vi "LauraMod_GlueFatLines.vi"(5 "Image Feed":T6=refnum, 7 "Template Path":path=path "C:/Users/Aerotech/Documents/BNL_ThermomechanicalStave/Utils/ConfigurationFiles_and_Templates/1_ModulePlacement", 8 "error in":errorcluster, 9 "um/pix resolution":dbl=1.58, 10 "Module corner coordinates":T2={"X [mm]"=-59.42477770816987, "Y [mm]"=4.341763392096446, "Z [mm] "=36.00000100000001}, 11 "XYZ Stage Control":refnum<k24>) -> (0 "error out":errorcluster={"status"=FALSE, "code"=1073676418, "source"="VISA Close in Alyssa_GlueFatLines.vi"}, 3 "XYZ .NET Refnum out":refnum<k24>)   [LabVIEW 2016]
uses:
  C:/Users/Aerotech/Documents/BNLStaveAssembly-blueprint/Bin/Aerotech.A3200.dll
  BNLStaveAssembly-blueprint/Bin/Aerotech.A3200.dll
  <vilib>/vision/Image Controls.llb/IMAQ Image.ctl
  <vilib>/LabVIEW Interface for Arduino/Type Defs/Arduino Resource.ctl
  <vilib>/LabVIEW Interface for Arduino/Type Defs/Board Type.ctl
  Utils/Controls/All_Enums/Enum_TypeDef_TapeType.ctl
  <vilib>/LabVIEW Interface for Arduino/Type Defs/Pin Mode.ctl
  <vilib>/Analysis/coordinate.llb/2D Cartesian Coordinate Rotation (Scalar).vi
  <vilib>/LabVIEW Interface for Arduino/LabVIEW Interface for Arduino.lvlib
  <vilib>/Analysis/NI_AALPro.lvlib
panel:
  out "main line speed":cluster{dbl, dbl, dbl}={21.85792349726776, 21.85792349726776, 21.85792349726776}
  in  "?":T1(tab)
  in  "Axis speeds (mm/s)":T3={"vX [mm]"=40.0, "vY [mm]"=40.0, "vZ [mm] "=40.0}
  in  "Home?":bool
  in  "Lowest Z Position":dbl=38.0
  out "Arduino Resource":T4={"VISA resource"="GlueCTRL", "Board Type"=enum."Uno", "Connection Type"=enum."USB / Serial", "Bytes Per Packet (15)"=15}
  in  "Digital I/O Pin":u8=7
  in  "Testing?":bool
  out "Difference camera/syringe in X":dbl=-133.03368290747076
  out "Difference camera/syringe in y":dbl=-2.170984960815403
  in  "Path to save collected images":path=path "C:/Users/Aerotech/cernbox/BNL/Stave Assembly Records/2017-06-12/3"
  in  "Estimate distance y":dbl
  in  "Estimate distance x":dbl=130.0
  in  "Lowest Z position Calibration":dbl=17.0
  in  "How many lines (actual x2)":i32=7
  in  "y dist (mm)":dbl=4.5
  out "bottom line speed":cluster{dbl, dbl, dbl}={32.78688524590164, 32.78688524590164, 32.78688524590164}
  out "mid line speed":cluster{dbl, dbl, dbl}={21.85792349726776, 21.85792349726776, 21.85792349726776}
  in  "Axial?":T7
  in  "glue time":dbl=2.25 format="%#_13g"
  out "top right speed":cluster{dbl, dbl, dbl}={5.46448087431694, 5.46448087431694, 5.46448087431694}
  out "top left speed":cluster{dbl, dbl, dbl}={21.85792349726776, 21.85792349726776, 21.85792349726776}
  out "Final Position":T8={"Final X"=-59.424942872475754, "Final Y"=8.342749448838399, "Final Z"=36.000300999844}
  out "Module Start":T8={"Final X"=-59.42477770816987, "Final Y"=4.341763392096446, "Final Z"=36.00000100000001}
  # "Overview: This takes a pattern of zeroes/ones (.csv file) as well as the start coordinates of the top left corner of a module and places dots of glue  \nRequirements: NI Arduino dependencies\nInstructions: Select a .csv file (ones indicate regions for glue) as well as a starting coordinate (this is default to the top left corner of the module spacer). You \ncan also input axis speeds (default to maximum) and module lengths and widths (default to 90 mm) which are the widths of the module to which you want to \nplace glue. Lastly, one can choose to Home the stage here and can select the lowest position in Z. The default is that the stage moves down 2-3 mm in Z \nwhile dispensing.  The Arduino inputs are default and simply allow the LabView program to drigger the Arduino (which sends a signal to the dispenser). The \nprogram signals to dispense air- all other parameters such as length of dispensing (default: 350 millisec), pressure (default: 48 psi), and vacuum pressure \n(default: 7.8 psi) are set on the dispenser itself. The defaults are highly recommended here."
  # "Positioning Inputs"
  # "Arduino Inputs"
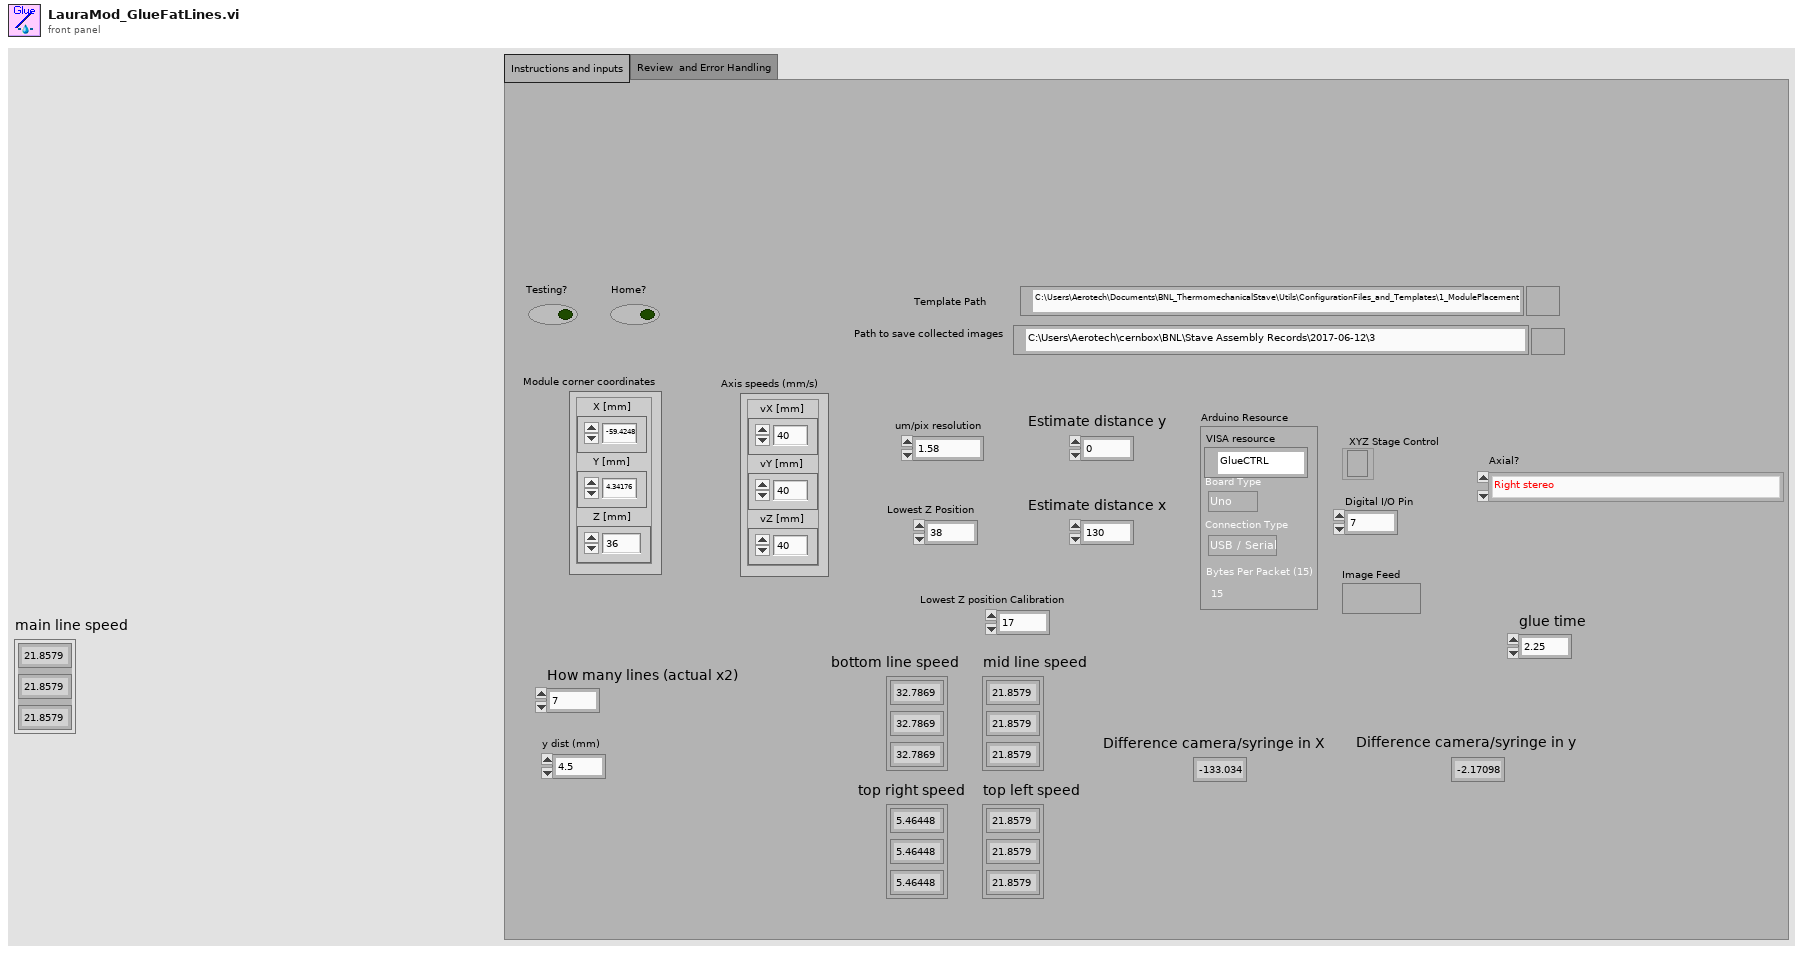
[diagram p1: front panel]
types:
  T1 = enum32{"Instructions and inputs", "Review  and Error Handling"}
  T2 = cluster{"X [mm]":dbl, "Y [mm]":dbl, "Z [mm] ":dbl}
  T3 = cluster{"vX [mm]":dbl, "vY [mm]":dbl, "vZ [mm] ":dbl}
  T4 = typedef "LabVIEW Interface for Arduino.lvlib/Arduino Resource.ctl" = cluster{"VISA resource":refnum<visa-resource-name>, "Board Type":T5, "Connection Type":enum8{"USB / Serial"}, "Bytes Per Packet (15)":u8}
  T5 = typedef "LabVIEW Interface for Arduino.lvlib/Board Type.ctl" = enum16{"Uno", "Dimuelanove w/Atmega 328", "Mega 2560"}
  T6 = typedef "IMAQ Image.ctl" = refnum<image>
  T7 = typedef "Enum_TypeDef_TapeType.ctl" = enum16{"Right stereo", "Left stereo", "Stereo (Sutcliffe Stave Core 9 LS)", "Stereo (Sutcliffe NP49-01-100 01-Mar-16)", "Stereo (Sutcliffe 21-Jun-18- Electrical)", "Axial (Sutcliffe NP49-01-100 01-Mar-16)", "Stereo (Sutcliffe Stave Core 8)"}
  T8 = cluster{"Final X":dbl, "Final Y":dbl, "Final Z":dbl}
  T9 = typedef "LabVIEW Interface for Arduino.lvlib/Pin Mode.ctl" = enum8{"Input", "Output"}
  T10 = cluster{dbl, "Y [mm]":dbl, "Lowest Z Position":dbl}
  T11 = cluster{"Final X":dbl, "Final Y":dbl, "vZ [mm]":dbl}
  T12 = cluster{dbl, "Final Y":dbl, "Lowest Z Position":dbl}
  T13 = cluster{"Final X":dbl, "Final Y":dbl, "Z [mm] ":dbl}
  T14 = cluster{"x out":dbl, "Final Y":dbl, "Lowest Z Position":dbl}
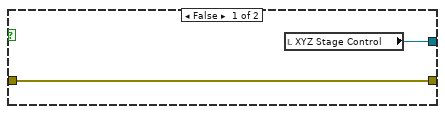
[diagram p2: hidden frame]
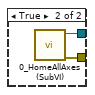
[diagram p3: hidden frame]
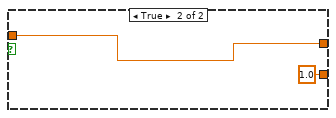
[diagram p5: hidden frame]
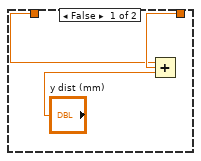
[diagram p6: hidden frame]
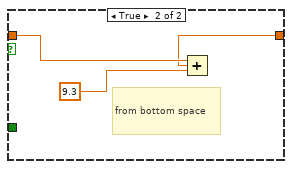
[diagram p7: hidden frame]
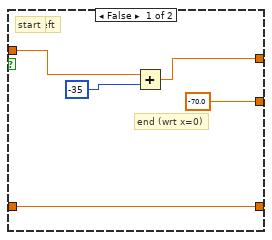
[diagram p8: hidden frame]
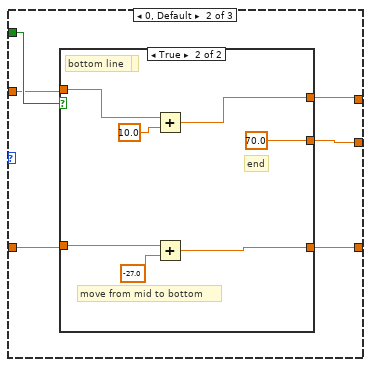
[diagram p9: hidden frame]
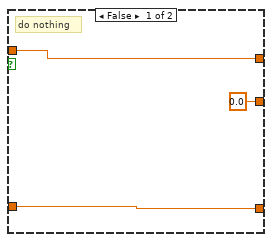
[diagram p10: hidden frame]
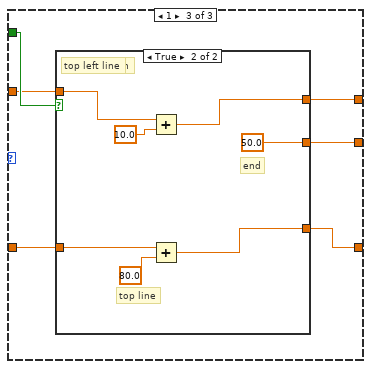
[diagram p11: hidden frame]
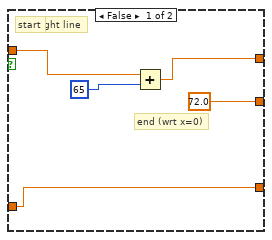
[diagram p12: hidden frame]
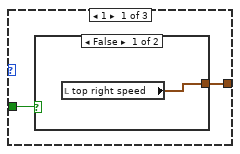
[diagram p13: hidden frame]
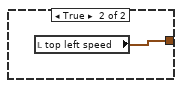
[diagram p14: hidden frame]
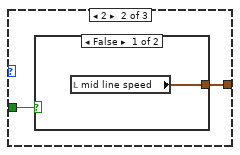
[diagram p15: hidden frame]
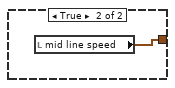
[diagram p16: hidden frame]
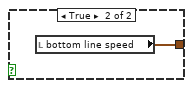
[diagram p17: hidden frame]
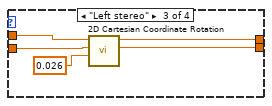
[diagram p19: hidden frame]
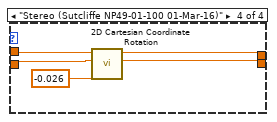
[diagram p20: hidden frame]
diagram:
  n1 = case shown="True" "Testing?" {
    tunnel: [w9 w11] -> w3
    tunnel: [w8 w10] -> w5
    tunnel: "error in" -> [w8 _]
    frame False {
      n2 = local read "XYZ Stage Control"() -> (w9:refnum<k24>)
    }
    frame True {
      n3 = case shown="False" "Home?" {
        tunnel: [w15 w21] -> w11
        tunnel: [w14 w20] -> w10
        frame False {
          w17 = string[] ["X", "Y", "Z"] ("Axes Names")
          n4 = call "Connect.vi"() -> ("error out"=w18:errorcluster, "controller"=w13:refnum<k24>)  [unwired: 10 in]
          n5 = call "EnableMultiple.vi"("error in (no error)"=w18, "axis names"=w17, "controller in"=w13) -> ("error out"=w19:errorcluster, "controller out"=w16:refnum<k24>)  [unwired: 7 in]
          n6 = call "GetCurrentXYZPosition (SubVI).vi"(".NET Refnum in - Device"=w16, "error in (no error)"=w19, "Axes Names"=w17) -> ("error out"=w14:errorcluster, ".NET Refnum out  - Device"=w15:refnum<k24>)  [unwired: 3 in, 4 out]
        }
        frame True {
          n7 = call "0_HomeAllAxes (SubVI).vi"() -> ("error out"=w20:errorcluster, "controller out"=w21:refnum<k24>)  [unwired: 8 in, 2 out]
        }
      }
    }
  }
  n8 = flat-sequence {
    tunnel: [w43] -> w7
    tunnel: w5 -> [w33]
    tunnel: w3 -> [w27]
    tunnel: [w196] -> w2
    tunnel: w7 -> [w199]
    tunnel: w2 -> [w349]
    tunnel: "Axial?" -> [w320]
    frame #0 {
      n9 = flat-sequence {
        tunnel: w33 -> [w57]
        tunnel: [w56] -> w28
        tunnel: w27 -> [w50]
        tunnel: w28 -> [w59]
        tunnel: [w58] -> w26
        tunnel: [w78] -> w30
        tunnel: w26 -> [w77]
        tunnel: w30 -> [w139]
        tunnel: [w137] -> w29
        tunnel: [w172] -> w31
        tunnel: w29 -> [w173]
        frame #0 {
          n10 = local read "Module corner coordinates"() -> (w52:T2)
          n11 = Unbundle(w52) -> ("X [mm]"=w49:dbl, "Y [mm]"=w46:dbl)  [unwired: 1 out]
          n12 = local read "Axis speeds (mm/s)"() -> (w55:T3)
          n13 = Add(x=w49, y=115.0) -> (x+y=w47:dbl)
          n14 = Bundle(w47, "Y [mm]"=w46, "Lowest Z Position"="Lowest Z Position") -> (w51:T10)  [unwired: 1 in]
          n15 = Bundle(w47, "Y [mm]"=w46, "Lowest Z Position"="Lowest Z Position") -> (w44:T10)  [unwired: 1 in]
          n16 = call "Go2XYZ (SubVI).vi"(".NET Refnum in"=w50, "Go to Coordinates"=w51, "Axis Speeds"=w55, "error in (no error)"=w57) -> (".NET Refnum out"=w54:refnum<k24>, "Final Position"=→"Final Position":T8, "error out"=w56:errorcluster)  [unwired: 7 in, 2 out]
          n17 = local write "Module corner coordinates"(w44) -> ()
          n18 = local write "XYZ Stage Control"(w54) -> ()
        }
        frame #1 {
          n19 = while {
            tunnel: w59 -> [w76]
            tunnel: [w72] -> w58
            stop <- w75 stop-if-true
            n20 = call "Lower glue mount"("error in (no error)"=w76) -> ("Move Z down"=w67:dbl, "Move Z up"=w66:dbl, "Accept current Z?"=w75:bool, "error out"=w73:errorcluster)  [unwired: 14 in, 1 out]
            n21 = local read "Module corner coordinates"() -> (w70:T2)
            n22 = local read "Lowest Z Position"() -> (w60:dbl)
            n23 = local read "Axis speeds (mm/s)"() -> (w74:T3)
            n24 = Add(x=w60, y=w67) -> (x+y=w64:dbl)
            n25 = local read "XYZ Stage Control"() -> (w62:refnum<k24>)
            n26 = Subtract(x=w64, y=w66) -> (x-y=w63:dbl)
            n27 = Unbundle(w70) -> ("X [mm]"=w69:dbl, "Y [mm]"=w68:dbl)  [unwired: 1 out]
            n28 = Bundle("X [mm]"=w69, "Y [mm]"=w68, w63) -> (w65:cluster{"X [mm]":dbl, "Y [mm]":dbl, dbl})  [unwired: 1 in]
            n29 = local write "Lowest Z Position"(w63) -> ()
            n30 = call "Go2XYZ (SubVI).vi"(".NET Refnum in"=w62, "Go to Coordinates"=w65, "Axis Speeds"=w74, "error in (no error)"=w73) -> (".NET Refnum out"=w71:refnum<k24>, "Final Position"=w61:T8, "error out"=w72:errorcluster)  [unwired: 7 in, 2 out]
            n31 = local write "Final Position"(w61) -> ()
            n32 = local write "XYZ Stage Control"(w71) -> ()
          }
        }
        frame #2 {
          n33 = call "Calibrate distance?"("error in (no error)"=w77) -> ("Calibrate distance?"=w79:bool, "error out"=w80:errorcluster)  [unwired: 16 in, 1 out]
          n34 = case shown="True" w79 {
            tunnel: w80 -> [w81 w83]
            tunnel: [w81 w84] -> w78
            frame False {
            }
            frame True {
              n35 = flat-sequence {
                tunnel: w83 -> [w86]
                tunnel: [w85] -> w82
                frame #0 {
                  n36 = local read "Final Position"() -> (w93:T8)
                  n37 = local read "Axis speeds (mm/s)"() -> (w89:T3)
                  n38 = local read "XYZ Stage Control"() -> (w88:refnum<k24>)
                  n39 = Unbundle(w93) -> ("Final X"=w91:dbl, "Final Y"=w92:dbl)  [unwired: 1 out]
                  n40 = Bundle("Final X"=w91, "Final Y"=w92, "vZ [mm]"=-20.0) -> (w95:T11)  [unwired: 1 in]
                  n41 = call "Go2XYZ (SubVI).vi"(".NET Refnum in"=w88, "Go to Coordinates"=w95, "Axis Speeds"=w89, "error in (no error)"=w86) -> (".NET Refnum out"=w87:refnum<k24>, "Final Position"=w90:T8, "error out"=w85:errorcluster)  [unwired: 7 in, 2 out]
                  n42 = local write "Final Position"(w90) -> ()
                  n43 = local write "XYZ Stage Control"(w87) -> ()
                }
              }
              n44 = while {
                tunnel: [w136] -> w84
                tunnel: w82 -> [w124]
                i -> [w121]
                stop <- w96 stop-if-true
                n45 = local read "Final Position"() -> (w98:T8)
                n46 = Unbundle(w98) -> ("Final X"=w103:dbl, "Final Y"=w101:dbl, "Final Z"=w102:dbl)
                n47 = local read "Testing?"() -> (w119:bool)
                n48 = local read "Axis speeds (mm/s)"() -> (w126:T3)
                n49 = local read "XYZ Stage Control"() -> (w122:refnum<k24>)
                n50 = Subtract(x=w101, y=220.0) -> (x-y=w99:dbl)
                n51 = Equal To 0?(x=w121) -> (x = 0?=w120:bool)
                n52 = And(x=w119, y=w120) -> (x .and. y?=w118:bool)
                n53 = Bundle("Final X"=w103, w99, "Final Z"=w102) -> (w104:cluster{"Final X":dbl, dbl, "Final Z":dbl})  [unwired: 1 in]
                n54 = call "CalibrateDistanceCameraSyringe.vi"("Path to save collected images"="Path to save collected images", "Image Feed"="Image Feed", "Off stave position"=w104, ".NET Refnum in"=w122, "Axis speeds (mm/s)"=w126, "Lowest Z Position"="Lowest Z position Calibration", "Estimate distance y"="Estimate distance y", "um/pix resolution"="um/pix resolution", "Estimate distance x"="Estimate distance x", "Template Path"="Template Path", "error in"=w124, "Testing?"=w118) -> ("XYZ .NET Refnum out"=w125:refnum<k24>, "error out"=w123:errorcluster, "X/Y difference (CAMERA - SYRINGE)"=w133:dbl[][])  [unwired: 1 in]
                n55 = local read "Difference camera/syringe in X"() -> (w108:dbl)
                n56 = local read "Difference camera/syringe in y"() -> (w105:dbl)
                n57 = local read "Lowest Z position Calibration"() -> (w110:dbl)
                n58 = call "Accept calibration?"("error in (no error)"=w123) -> ("Change in lowest Z"=w112:dbl, "Change in distance Y estimate"=w113:dbl, "Change in distance X estimate"=w114:dbl, "Accept the distance syringe/camera?"=w96:bool, "error out"=w136:errorcluster)  [unwired: 13 in, 1 out]
                n59 = local write "XYZ Stage Control"(w125) -> ()
                n60 = Index Array(array=w133, index (row) #1=0 ("index (row)"), index (col) #1=0 ("disabled index (col)"), index (row) #2=0 ("index (row)"), index (col) #2=1 ("disabled index (col)")) -> (element #1=→"Difference camera/syringe in X":dbl, element #2=→"Difference camera/syringe in y":dbl)
                n61 = Add(x=w108, y=w114) -> (x+y=w107:dbl)
                n62 = Add(x=w105, y=w113) -> (x+y=w106:dbl)
                n63 = Add(x=w110, y=w112) -> (x+y=w111:dbl)
                n64 = local write "Lowest Z position Calibration"(w111) -> ()
                n65 = local write "Difference camera/syringe in X"(w107) -> ()
                n66 = local write "Difference camera/syringe in y"(w106) -> ()
              }
            }
          }
        }
        frame #3 {
          n67 = flat-sequence {
            tunnel: w139 -> [w149]
            tunnel: [w146] -> w138
            tunnel: [w159] -> w137
            tunnel: w138 -> [w160]
            frame #0 {
              n68 = local read "Module corner coordinates"() -> (w158:T2)
              n69 = local read "Difference camera/syringe in y"() -> (w154:dbl)
              n70 = local read "Difference camera/syringe in X"() -> (w155:dbl)
              n71 = Unbundle By Name(w158) -> ("X [mm]"=w145:dbl, "Y [mm]"=w157:dbl)  [unwired: 1 out]
              n72 = Subtract(x=w157, y=w154) -> (x-y=w142:dbl)
              n73 = Subtract(x=w145, y=136.0) -> (x-y=w143:dbl)
              n74 = local read "Axis speeds (mm/s)"() -> (w150:T3)
              n75 = local read "XYZ Stage Control"() -> (w151:refnum<k24>)
              n76 = Subtract(x=w142, y=83.0) -> (x-y=w140:dbl)
              n77 = Subtract(x=w143, y=w155) -> (x-y=w156:dbl)
              n78 = Bundle(w156, w140, "index (row)"=-20.0) -> (w148:cluster{dbl, dbl, "index (row)":dbl})  [unwired: 1 in]
              n79 = call "Go2XYZ (SubVI).vi"(".NET Refnum in"=w151, "Go to Coordinates"=w148, "Axis Speeds"=w150, "error in (no error)"=w149) -> (".NET Refnum out"=w152:refnum<k24>, "Final Position"=w153:T8, "error out"=w146:errorcluster)  [unwired: 7 in, 2 out]
              n80 = local write "XYZ Stage Control"(w152) -> ()
              n81 = local write "Module corner coordinates"(w153) -> ()
            }
            frame #1 {
              n82 = local read "Module corner coordinates"() -> (w165:T2)
              n83 = local read "Lowest Z Position"() -> (w168:dbl)
              n84 = local read "Axis speeds (mm/s)"() -> (w162:T3)
              n85 = local read "XYZ Stage Control"() -> (w161:refnum<k24>)
              n86 = Unbundle(w165) -> ("X [mm]"=w166:dbl, "Y [mm]"=w167:dbl)  [unwired: 1 out]
              n87 = Subtract(x=w168, y=2.0) -> (x-y=w170:dbl)
              n88 = Bundle("X [mm]"=w166, "Y [mm]"=w167, w170) -> (w171:cluster{"X [mm]":dbl, "Y [mm]":dbl, dbl})  [unwired: 1 in]
              n89 = call "Go2XYZ (SubVI).vi"(".NET Refnum in"=w161, "Go to Coordinates"=w171, "Axis Speeds"=w162, "error in (no error)"=w160) -> (".NET Refnum out"=w163:refnum<k24>, "Final Position"=w164:T8, "error out"=w159:errorcluster)  [unwired: 7 in, 2 out]
              n90 = local write "XYZ Stage Control"(w163) -> ()
              n91 = local write "Module corner coordinates"(w164) -> ()
            }
          }
        }
        frame #4 {
          n92 = while {
            tunnel: w173 -> [w187]
            tunnel: [w189] -> w172
            stop <- w174 stop-if-true
            n93 = local read "Module corner coordinates"() -> (w186:T2)
            n94 = call "Ready to glue?"("error in (no error)"=w187) -> ("Move in Z"=w183:dbl, "Move in Y"=w184:dbl, "Move in X"=w185:dbl, "Oh yeah! Reset Arduino and go!"=w174:bool, "error out"=w188:errorcluster)  [unwired: 13 in, 1 out]
            n95 = local read "Axis speeds (mm/s)"() -> (w192:T3)
            n96 = local read "XYZ Stage Control"() -> (w190:refnum<k24>)
            n97 = Unbundle(w186) -> ("X [mm]"=w182:dbl, "Y [mm]"=w181:dbl, "Z [mm]"=w180:dbl)
            n98 = Add(x=w182, y=w185) -> (x+y=w177:dbl)
            n99 = Add(x=w181, y=w184) -> (x+y=w179:dbl)
            n100 = Add(x=w180, y=w183) -> (x+y=w178:dbl)
            n101 = Bundle(w177, w179, w178) -> (w176:cluster{dbl, dbl, dbl})  [unwired: 1 in]
            n102 = call "Go2XYZ (SubVI).vi"(".NET Refnum in"=w190, "Go to Coordinates"=w176, "Axis Speeds"=w192, "error in (no error)"=w188) -> (".NET Refnum out"=w191:refnum<k24>, "Final Position"=w175:T8, "error out"=w189:errorcluster)  [unwired: 7 in, 2 out]
            "Module Start" <- w175
            n103 = local write "Final Position"(w175) -> ()
            n104 = local write "XYZ Stage Control"(w191) -> ()
            n105 = local write "Module corner coordinates"(w175) -> ()
          }
        }
      }
      n106 = local read "Digital I/O Pin"() -> (w32:u8)
      n107 = local read "glue time"() -> (w24:dbl)
      n108 = call <vilib>:"Init.vi"("VISA resource"=refnum<visa-resource-name> "GlueCTRL", "error in"=w31) -> ("Arduino Resource"=w35:T4, "error out"=w36:errorcluster)  [unwired: 16 in]
      "Arduino Resource" <- w35
      n109 = call <vilib>:"Set Digital Pin Mode.vi"("Arduino Resource"=w35, "Digital I/O Pin"="Digital I/O Pin", "Pin Mode (Input)"=Pin_Mode."Output", "error in"=w36) -> ("Arduino Resource"=w39:T4, "error out"=w40:errorcluster)  [unwired: 10 in]
      n110 = Divide(x=80.0 ("vX [mm]"), y=w24) -> (x/y=w23:dbl)
      n111 = call <vilib>:"Digital Write Pin.vi"("Arduino Resource"=w39, "Digital I/O Pin (0)"=w32, "Value (0)"=u8 0, "error in"=w40) -> ("Arduino Resource"=w34:T4, "error out"=w43:errorcluster)  [unwired: 10 in]
      n112 = Bundle(w23, w23, w23) -> (→"main line speed":cluster{dbl, dbl, dbl})  [unwired: 1 in]
      n113 = local write "Arduino Resource"(w34) -> ()
    }
    frame #1 {
      n114 = local read "Module Start"() -> (w198:T8)
      n115 = Unbundle By Name(w198) -> ("Final X"=w193:dbl, "Final Y"=w194:dbl, "Final Z"=w197:dbl)
      n116 = for {
        N: "How many lines (actual x2)" -> [_]
        tunnel: w199 -> [w211]
        tunnel: [w210] -> w196
        shift-right: [w209] -> _
        shift-left: w194 -> [w201]
        tunnel: w197 -> [w208]
        shift-right: [w207] -> _
        shift-left: w193 -> [w202]
        i -> [w205]
        n117 = Equal?(x=w205, y=2) -> (x = y?=w203:bool)
        n118 = Equal To 0?(x=w205) -> (x = 0?=w204:bool)
        n119 = for {
          N: 2 -> [_]
          tunnel: w211 -> [w233]
          tunnel: [w231] -> w210
          shift-right: [w230] -> w209
          shift-left: w201 -> [w221]
          tunnel: w208 -> [w220]
          tunnel: w202 -> [w222]
          tunnel: [w218] -> w207
          tunnel: w204 -> [w213]
          tunnel: w203 -> [w212]
          i -> [w219]
          n120 = flat-sequence {
            tunnel: w233 -> [w251]
            tunnel: [w236] -> w228
            tunnel: [w251] -> w227
            tunnel: [w239] -> w226
            tunnel: [w238] -> w225
            tunnel: [w250] -> w224
            tunnel: [w239] -> w223
            tunnel: w222 -> [w237]
            tunnel: w221 -> [w240]
            tunnel: w220 -> [w250]
            tunnel: w219 -> [w244]
            tunnel: w213 -> [w243]
            tunnel: w212 -> [w242]
            tunnel: [w279] -> w216
            tunnel: [w280] -> w215
            tunnel: [w281] -> w214
            tunnel: w223 -> [w281]
            tunnel: w224 -> [w278]
            tunnel: w225 -> [w271]
            tunnel: w226 -> [w270]
            tunnel: w227 -> [w274]
            tunnel: w228 -> [w279]
            tunnel: [w299] -> w235
            tunnel: [w298] -> w234
            tunnel: [w297] -> w232
            tunnel: [w290] -> w229
            tunnel: w216 -> [w287]
            tunnel: w215 -> [w289]
            tunnel: w214 -> [w290]
            tunnel: [w287] -> w217
            tunnel: [w319] -> w231
            tunnel: w232 -> [w307]
            tunnel: w234 -> [w318]
            tunnel: w235 -> [w316]
            tunnel: [w306] -> w230
            tunnel: w229 -> [w306]
            tunnel: [w305] -> w218
            tunnel: w217 -> [w305]
            frame #0 {
              # "line length"
              n121 = Equal To 0?(x=w244) -> (x = 0?=w241:bool)
              n122 = case shown="False" w241 {
                tunnel: [0.0 1.0] -> w246
                tunnel: [w253 w256] -> w238
                tunnel: w237 -> [w254 w256]
                frame False {
                  # "start @ end of line"
                  n123 = Add(x=w254, y=80 ("x")) -> (x+y=w253:dbl)
                }
                frame True {
                }
              }
              n124 = And(x=w241, y=w243) -> (x .and. y?=w245:bool)
              n125 = And(x=w241, y=w242) -> (x .and. y?=w249:bool)
              n126 = case shown="False" w245 {
                tunnel: w240 -> [w259 w269]
                tunnel: [w260 w268] -> w239
                tunnel: w249 -> [w258 _]
                frame False {
                  n127 = case shown="True" w258 {
                    tunnel: [w263 w264] -> w260
                    tunnel: w259 -> [w261 w266]
                    frame False {
                      n128 = Add(x=w261, y="y dist (mm)") -> (x+y=w263:dbl)
                    }
                    frame True {
                      # "center space"
                      n129 = Add(x=w266, y=11.0) -> (x+y=w264:dbl)
                    }
                  }
                }
                frame True {
                  # "from bottom space"
                  n130 = Add(x=w269, y=9.3) -> (x+y=w268:dbl)
                }
              }
              n131 = Multiply(x=80, y=w246) -> (x*y=w247:dbl)
              n132 = Add(x=w237, y=w247) -> (x+y=w236:dbl)
            }
            frame #1 {
              n133 = local read "Axis speeds (mm/s)"() -> (w276:T3)
              n134 = local read "XYZ Stage Control"() -> (w273:refnum<k24>)
              n135 = Bundle("Final X"=w271, w270, "Final Z"=w278) -> (w277:cluster{"Final X":dbl, dbl, "Final Z":dbl})  [unwired: 1 in]
              n136 = call "Go2XYZ (SubVI).vi"(".NET Refnum in"=w273, "Go to Coordinates"=w277, "Axis Speeds"=w276, "error in (no error)"=w274) -> (".NET Refnum out"=w272:refnum<k24>, "Final Position"=w275:T8, "error out"=w280:errorcluster)  [unwired: 7 in, 2 out]
              n137 = local write "Final Position"(w275) -> ()
              n138 = local write "XYZ Stage Control"(w272) -> ()
            }
            frame #2 {
              n139 = local read "Lowest Z Position"() -> (w296:dbl)
              n140 = local read "Final Position"() -> (w291:T8)
              n141 = local read "main line speed"() -> (w286:cluster{dbl, dbl, dbl})
              n142 = Unbundle(w286) -> (w285:dbl, w284:dbl)  [unwired: 1 out]
              n143 = Bundle(w285, "x"=1.04, w284) -> (w283:cluster{dbl, "x":dbl, dbl})  [unwired: 1 in]
              n144 = local read "Arduino Resource"() -> (w300:T4)
              n145 = local read "Digital I/O Pin"() -> (w299:u8)
              n146 = Unbundle(w291) -> ("Final Y"=w288:dbl)  [unwired: 2 out]
              n147 = local read "XYZ Stage Control"() -> (w294:refnum<k24>)
              n148 = Bundle(w287, "Final Y"=w288, "Lowest Z Position"=w296) -> (w293:T12)  [unwired: 1 in]
              n149 = call "Go2XYZ (SubVI).vi"(".NET Refnum in"=w294, "Go to Coordinates"=w293, "Axis Speeds"=w283) -> (".NET Refnum out"=w295:refnum<k24>, "Final Position"=w292:T8)  [unwired: 8 in, 3 out]
              n150 = local write "Final Position"(w292) -> ()
              n151 = call <vilib>:"Digital Write Pin.vi"("Arduino Resource"=w300, "Digital I/O Pin (0)"=w299, "Value (0)"=u8 1, "error in"=w289) -> ("Arduino Resource"=w298:T4, "error out"=w297:errorcluster)  [unwired: 10 in]
              n152 = local write "Arduino Resource"(w298) -> ()
              n153 = local write "XYZ Stage Control"(w295) -> ()
            }
            frame #3 {
              n154 = local read "Final Position"() -> (w314:T8)
              n155 = local read "Module corner coordinates"() -> (w313:T2)
              n156 = call <vilib>:"Digital Write Pin.vi"("Arduino Resource"=w318, "Digital I/O Pin (0)"=w316, "Value (0)"=u8 0, "error in"=w307) -> ("Arduino Resource"=w315:T4, "error out"=w319:errorcluster)  [unwired: 10 in]
              n157 = Unbundle(w314) -> ("Final X"=w304:dbl, "Final Y"=w303:dbl)  [unwired: 1 out]
              n158 = local write "Arduino Resource"(w315) -> ()
              n159 = Unbundle(w313) -> ("Z [mm]"=w312:dbl)  [unwired: 2 out]
              n160 = local read "XYZ Stage Control"() -> (w309:refnum<k24>)
              n161 = local read "Axis speeds (mm/s)"() -> (w310:T3)
              n162 = Bundle("Final X"=w304, "Final Y"=w303, "Z [mm]"=w312) -> (w311:T13)  [unwired: 1 in]
              n163 = call "Go2XYZ (SubVI).vi"(".NET Refnum in"=w309, "Go to Coordinates"=w311, "Axis Speeds"=w310) -> (".NET Refnum out"=w302:refnum<k24>, "Final Position"=w308:T8)  [unwired: 8 in, 3 out]
              n164 = local write "Final Position"(w308) -> ()
              n165 = local write "XYZ Stage Control"(w302) -> ()
            }
          }
        }
      }
    }
    frame #2 {
      n166 = local read "glue time"() -> (w334:dbl)
      n167 = local read "Module Start"() -> (w350:T8)
      n168 = Unbundle By Name(w350) -> ("Final X"=w338:dbl, "Final Y"=w339:dbl, "Final Z"=w348:dbl)
      n169 = Divide(x=35.0 ("vX [mm]"), y=w334) -> (x/y=w332:dbl)
      n170 = Divide(x=60.0 ("vX [mm]"), y="glue time") -> (x/y=w333:dbl)
      n171 = Bundle(w332, w332, w332) -> (→"mid line speed":cluster{dbl, dbl, dbl})  [unwired: 1 in]
      n172 = Bundle(w333, w333, w333) -> (→"bottom line speed":cluster{dbl, dbl, dbl})  [unwired: 1 in]
      n173 = for {
        N: 3 -> [_]
        tunnel: w349 -> [w368]
        tunnel: [w367] -> w342
        shift-right: [w365] -> _
        shift-left: w339 -> [w366]
        tunnel: w348 -> [w364]
        shift-right: [w363] -> _
        shift-left: w338 -> [w362]
        tunnel: w320 -> [w353]
        tunnel: w320 -> [w352]
        tunnel: w320 -> [w351]
        i -> [w357]
        n174 = Equal?(x=w357, y=2) -> (x = y?=w354:bool)
        n175 = Equal?(x=w357, y=1) -> (x = y?=w355:bool)
        n176 = Equal?(x=w357, y=0) -> (x = y?=w356:bool)
        n177 = for {
          N: 2 -> [_]
          tunnel: w368 -> [w403]
          tunnel: [w401] -> w367
          shift-right: [w400] -> w365
          shift-left: w366 -> [w392]
          tunnel: w364 -> [w391]
          tunnel: w362 -> [w384]
          tunnel: [w389] -> w363
          tunnel: w356 -> [w383]
          tunnel: w355 -> [w382]
          tunnel: w354 -> [w373]
          tunnel: w353 -> [w371]
          tunnel: w352 -> [w370]
          tunnel: w351 -> [w369]
          i -> [w390]
          n178 = flat-sequence {
            tunnel: w403 -> [w418]
            tunnel: [w416] -> w398
            tunnel: [w418] -> w397
            tunnel: [w408] -> w396
            tunnel: [w409] -> w395
            tunnel: [w417] -> w394
            tunnel: [w408] -> w393
            tunnel: w384 -> [w407]
            tunnel: w392 -> [w406]
            tunnel: w391 -> [w417]
            tunnel: w390 -> [w414]
            tunnel: w383 -> [w413]
            tunnel: w382 -> [w412]
            tunnel: w373 -> [w411]
            tunnel: [w405] -> w381
            tunnel: [w404] -> w380
            tunnel: [w404] -> w374
            tunnel: [w488] -> w387
            tunnel: [w487] -> w386
            tunnel: [w486] -> w385
            tunnel: w393 -> [w486]
            tunnel: w394 -> [w485]
            tunnel: w395 -> [w479]
            tunnel: w396 -> [w478]
            tunnel: w397 -> [w482]
            tunnel: w398 -> [w488]
            tunnel: w381 -> [w474]
            tunnel: w380 -> [w473]
            tunnel: [w474] -> w379
            tunnel: [w473] -> w378
            tunnel: [w472] -> w375
            tunnel: w374 -> [w472]
            tunnel: w371 -> [w471]
            tunnel: [w533] -> w402
            tunnel: [w526] -> w399
            tunnel: w387 -> [w524]
            tunnel: w386 -> [w525]
            tunnel: w385 -> [w526]
            tunnel: [w524] -> w388
            tunnel: w379 -> [w519]
            tunnel: w378 -> [w518]
            tunnel: [w519] -> w377
            tunnel: [w518] -> w376
            tunnel: w373 -> [w517]
            tunnel: w375 -> [w516]
            tunnel: [w516] -> w372
            tunnel: w370 -> [w515]
            tunnel: [w596] -> w401
            tunnel: w402 -> [w589]
            tunnel: [w588] -> w400
            tunnel: w399 -> [w588]
            tunnel: [w587] -> w389
            tunnel: w388 -> [w587]
            tunnel: w377 -> [w581]
            tunnel: w376 -> [w580]
            tunnel: w373 -> [w579]
            tunnel: w372 -> [w578]
            tunnel: w369 -> [w577]
            frame #0 {
              # "where to move"
              n179 = Build Array(w413, w412, w411) -> (w415:bool[])
              n180 = Equal To 0?(x=w414) -> (x = 0?=w404:bool)
              n181 = Boolean Array To Number(Boolean array=w415) -> (number=w405:u32)
              n182 = case shown="2" w405 {
                tunnel: w404 -> [w419 w438 w458]
                tunnel: w407 -> [w423 w437 w457]
                tunnel: w406 -> [w424 w442 w456]
                tunnel: [w422 w439 w455] -> w408
                tunnel: [w421 w440 w454] -> w410
                tunnel: [w420 w441 w453] -> w409
                frame 2 {
                  n183 = case shown="True" w419 {
                    tunnel: [w428 w435] -> w420
                    tunnel: w423 -> [w429 w436]
                    tunnel: [-70.0 -27.0 ("y")] -> w421
                    tunnel: w424 -> [w425 w431]
                    tunnel: [w425 w430] -> w422
                    frame False {
                      # "mid left"
                      # "end (wrt x=0)"
                      # "start"
                      n184 = Add(x=w429, y=-35 ("x")) -> (x+y=w428:dbl)
                    }
                    frame True {
                      # "move down to mid line"
                      # "end"
                      # "middle right"
                      # "start position wrt previous x"
                      n185 = Add(x=w436, y=8.0) -> (x+y=w435:dbl)
                      n186 = Add(x=w431, y=-50.0) -> (x+y=w430:dbl)
                    }
                  }
                }
                frame 0, Default {
                  n187 = case shown="True" w438 {
                    tunnel: [w444 w451] -> w441
                    tunnel: w437 -> [w444 w452]
                    tunnel: [0.0 ("y") 70.0 ("y")] -> w440
                    tunnel: w442 -> [w445 w447]
                    tunnel: [w445 w446] -> w439
                    frame False {
                      # "do nothing"
                    }
                    frame True {
                      # "move from mid to bottom"
                      # "end"
                      # "bottom line"
                      # "start position"
                      n188 = Add(x=w452, y=10.0) -> (x+y=w451:dbl)
                      n189 = Add(x=w447, y=-27.0) -> (x+y=w446:dbl)
                    }
                  }
                }
                frame 1 {
                  n190 = case shown="True" w458 {
                    tunnel: [w462 w469] -> w453
                    tunnel: w457 -> [w463 w470]
                    tunnel: [72.0 50.0 ("y")] -> w454
                    tunnel: w456 -> [w459 w465]
                    tunnel: [w459 w464] -> w455
                    frame False {
                      # "top right line"
                      # "end (wrt x=0)"
                      # "start"
                      n191 = Add(x=w463, y=65 ("x")) -> (x+y=w462:dbl)
                    }
                    frame True {
                      # "top line"
                      # "end"
                      # "top left line"
                      # "start position"
                      n192 = Add(x=w470, y=10.0) -> (x+y=w469:dbl)
                      n193 = Add(x=w465, y=80.0) -> (x+y=w464:dbl)
                    }
                  }
                }
              }
              n194 = Add(x=w407, y=w410) -> (x+y=w416:dbl)
            }
            frame #1 {
              n195 = case shown="\"Stereo (Sutcliffe 21-Jun-18- Electrical)\"" w471 {
                tunnel: w479 -> [w502 w504 w509 w512]
                tunnel: w478 -> [w501 w503 w508 w511]
                tunnel: [w502 w504 w506 w514] -> w477
                tunnel: [w501 w503 w505 w513] -> w476
                frame "Right stereo", Default {
                }
                frame "Stereo (Sutcliffe 21-Jun-18- Electrical)" {
                }
                frame "Left stereo" {
                  n196 = call-poly <vilib>:"2D Cartesian Coordinate Rotation.vi"("theta"=0.026, "y"=w508, "x"=w509) -> ("y out"=w505:dbl, "x out"=w506:dbl)  [unwired: 6 in, 1 out]
                }
                frame "Stereo (Sutcliffe NP49-01-100 01-Mar-16)" {
                  n197 = call-poly <vilib>:"2D Cartesian Coordinate Rotation.vi"("theta"=-0.026, "y"=w511, "x"=w512) -> ("y out"=w513:dbl, "x out"=w514:dbl)  [unwired: 6 in, 1 out]
                }
              }
              n198 = case shown="0, Default" w474 {
                tunnel: w473 -> [w490 w494 w498]
                tunnel: [w489 w493 w497] -> w475
                frame 1 {
                  n199 = case shown="False" w490 {
                    tunnel: [w491 w492] -> w489
                    frame False {
                      n200 = local read "top right speed"() -> (w491:cluster{dbl, dbl, dbl})
                    }
                    frame True {
                      n201 = local read "top left speed"() -> (w492:cluster{dbl, dbl, dbl})
                    }
                  }
                }
                frame 2 {
                  n202 = case shown="False" w494 {
                    tunnel: [w495 w496] -> w493
                    frame False {
                      n203 = local read "mid line speed"() -> (w495:cluster{dbl, dbl, dbl})
                    }
                    frame True {
                      n204 = local read "mid line speed"() -> (w496:cluster{dbl, dbl, dbl})
                    }
                  }
                }
                frame 0, Default {
                  n205 = case shown="False" w498 {
                    tunnel: [w499 w500] -> w497
                    frame False {
                      n206 = local read "bottom line speed"() -> (w499:cluster{dbl, dbl, dbl})
                    }
                    frame True {
                      n207 = local read "bottom line speed"() -> (w500:cluster{dbl, dbl, dbl})
                    }
                  }
                }
              }
              n208 = Bundle("x out"=w477, "y out"=w476, "Final Z"=w485) -> (w484:cluster{"x out":dbl, "y out":dbl, "Final Z":dbl})  [unwired: 1 in]
              n209 = local read "XYZ Stage Control"() -> (w481:refnum<k24>)
              n210 = call "Go2XYZ (SubVI).vi"(".NET Refnum in"=w481, "Go to Coordinates"=w484, "Axis Speeds"=w475, "error in (no error)"=w482) -> (".NET Refnum out"=w480:refnum<k24>, "Final Position"=w483:T8, "error out"=w487:errorcluster)  [unwired: 7 in, 2 out]
              n211 = local write "Final Position"(w483) -> ()
              n212 = local write "XYZ Stage Control"(w480) -> ()
            }
            frame #2 {
              n213 = local read "Final Position"() -> (w527:T8)
              n214 = case shown="True" w517 {
                tunnel: [w536 w542] -> w533
                tunnel: w525 -> [w535 w541]
                tunnel: w516 -> [_ w540]
                frame False {
                  n215 = local read "Arduino Resource"() -> (w539:T4)
                  n216 = local read "Digital I/O Pin"() -> (w538:u8)
                  n217 = call <vilib>:"Digital Write Pin.vi"("Arduino Resource"=w539, "Digital I/O Pin (0)"=w538, "Value (0)"=u8 1, "error in"=w535) -> ("Arduino Resource"=w537:T4, "error out"=w536:errorcluster)  [unwired: 10 in]
                  n218 = local write "Arduino Resource"(w537) -> ()
                }
                frame True {
                  n219 = case shown="True" w540 {
                    tunnel: [w543 w545] -> w542
                    tunnel: w541 -> [w543 w544]
                    frame False {
                    }
                    frame True {
                      n220 = local read "Arduino Resource"() -> (w548:T4)
                      n221 = local read "Digital I/O Pin"() -> (w547:u8)
                      n222 = call <vilib>:"Digital Write Pin.vi"("Arduino Resource"=w548, "Digital I/O Pin (0)"=w547, "Value (0)"=u8 1, "error in"=w544) -> ("Arduino Resource"=w546:T4, "error out"=w545:errorcluster)  [unwired: 10 in]
                      n223 = local write "Arduino Resource"(w546) -> ()
                    }
                  }
                }
              }
              n224 = Unbundle(w527) -> ("Final Y"=w523:dbl)  [unwired: 2 out]
              n225 = case shown="\"Stereo (Sutcliffe 21-Jun-18- Electrical)\"" w515 {
                tunnel: w524 -> [w563 w568 w571 w575]
                tunnel: w523 -> [w562 w567 w570 w574]
                tunnel: [w563 w565 w573 w575] -> w521
                tunnel: [w562 w564 w572 w574] -> w522
                frame "Right stereo", Default {
                }
                frame "Left stereo" {
                  n226 = call-poly <vilib>:"2D Cartesian Coordinate Rotation.vi"("theta"=0.026, "y"=w567, "x"=w568) -> ("y out"=w564:dbl, "x out"=w565:dbl)  [unwired: 6 in, 1 out]
                }
                frame "Stereo (Sutcliffe NP49-01-100 01-Mar-16)" {
                  n227 = call-poly <vilib>:"2D Cartesian Coordinate Rotation.vi"("theta"=-0.026, "y"=w570, "x"=w571) -> ("y out"=w572:dbl, "x out"=w573:dbl)  [unwired: 6 in, 1 out]
                }
                frame "Stereo (Sutcliffe 21-Jun-18- Electrical)" {
                }
              }
              n228 = case shown="2" w519 {
                tunnel: w518 -> [w551 w555 w559]
                tunnel: [w550 w554 w558] -> w520
                frame 1 {
                  n229 = case shown="False" w551 {
                    tunnel: [w552 w553] -> w550
                    frame False {
                      n230 = local read "top right speed"() -> (w552:cluster{dbl, dbl, dbl})
                    }
                    frame True {
                      n231 = local read "top left speed"() -> (w553:cluster{dbl, dbl, dbl})
                    }
                  }
                }
                frame 2 {
                  n232 = case shown="False" w555 {
                    tunnel: [w556 w557] -> w554
                    frame False {
                      n233 = local read "mid line speed"() -> (w556:cluster{dbl, dbl, dbl})
                    }
                    frame True {
                      n234 = local read "mid line speed"() -> (w557:cluster{dbl, dbl, dbl})
                    }
                  }
                }
                frame 0, Default {
                  n235 = case shown="False" w559 {
                    tunnel: [w560 w561] -> w558
                    frame False {
                      n236 = local read "bottom line speed"() -> (w560:cluster{dbl, dbl, dbl})
                    }
                    frame True {
                      n237 = local read "bottom line speed"() -> (w561:cluster{dbl, dbl, dbl})
                    }
                  }
                }
              }
              n238 = local read "Lowest Z Position"() -> (w532:dbl)
              n239 = local read "XYZ Stage Control"() -> (w530:refnum<k24>)
              n240 = Bundle("x out"=w521, "Final Y"=w522, "Lowest Z Position"=w532) -> (w529:T14)  [unwired: 1 in]
              n241 = call "Go2XYZ (SubVI).vi"(".NET Refnum in"=w530, "Go to Coordinates"=w529, "Axis Speeds"=w520) -> (".NET Refnum out"=w531:refnum<k24>, "Final Position"=w528:T8)  [unwired: 8 in, 3 out]
              n242 = local write "XYZ Stage Control"(w531) -> ()
              n243 = local write "Final Position"(w528) -> ()
            }
            frame #3 {
              n244 = case shown="True" w579 {
                tunnel: [w598 w605] -> w596
                tunnel: w589 -> [w597 w604]
                tunnel: w578 -> [_ w603]
                frame False {
                  n245 = local read "Digital I/O Pin"() -> (w599:u8)
                  n246 = local read "Arduino Resource"() -> (w600:T4)
                  n247 = call <vilib>:"Digital Write Pin.vi"("Arduino Resource"=w600, "Digital I/O Pin (0)"=w599, "Value (0)"=u8 0, "error in"=w597) -> ("Arduino Resource"=w601:T4, "error out"=w598:errorcluster)  [unwired: 10 in]
                  n248 = local write "Arduino Resource"(w601) -> ()
                }
                frame True {
                  n249 = case shown="True" w603 {
                    tunnel: [w606 w612] -> w605
                    tunnel: w604 -> [w606 w609]
                    frame False {
                    }
                    frame True {
                      n250 = local read "Digital I/O Pin"() -> (w607:u8)
                      n251 = local read "Arduino Resource"() -> (w608:T4)
                      n252 = call <vilib>:"Digital Write Pin.vi"("Arduino Resource"=w608, "Digital I/O Pin (0)"=w607, "Value (0)"=u8 0, "error in"=w609) -> ("Arduino Resource"=w610:T4, "error out"=w612:errorcluster)  [unwired: 10 in]
                      n253 = local write "Arduino Resource"(w610) -> ()
                    }
                  }
                }
              }
              n254 = local read "Final Position"() -> (w595:T8)
              n255 = local read "Module Start"() -> (w594:T8)
              n256 = Unbundle(w595) -> ("Final X"=w585:dbl, "Final Y"=w586:dbl)  [unwired: 1 out]
              n257 = Unbundle(w594) -> ("Final Z"=w593:dbl)  [unwired: 2 out]
              n258 = case shown="\"Stereo (Sutcliffe 21-Jun-18- Electrical)\"" w577 {
                tunnel: w585 -> [w626 w631 w634 w638]
                tunnel: w586 -> [w625 w630 w633 w637]
                tunnel: [w626 w628 w636 w638] -> w584
                tunnel: [w625 w627 w635 w637] -> w583
                frame "Right stereo", Default {
                }
                frame "Left stereo" {
                  n259 = call-poly <vilib>:"2D Cartesian Coordinate Rotation.vi"("theta"=0.026, "y"=w630, "x"=w631) -> ("y out"=w627:dbl, "x out"=w628:dbl)  [unwired: 6 in, 1 out]
                }
                frame "Stereo (Sutcliffe NP49-01-100 01-Mar-16)" {
                  n260 = call-poly <vilib>:"2D Cartesian Coordinate Rotation.vi"("theta"=-0.026, "y"=w633, "x"=w634) -> ("y out"=w635:dbl, "x out"=w636:dbl)  [unwired: 6 in, 1 out]
                }
                frame "Stereo (Sutcliffe 21-Jun-18- Electrical)" {
                }
              }
              n261 = local read "XYZ Stage Control"() -> (w591:refnum<k24>)
              n262 = case shown="0, Default" w581 {
                tunnel: w580 -> [w614 w618 w622]
                tunnel: [w613 w617 w621] -> w582
                frame 1 {
                  n263 = case shown="False" w614 {
                    tunnel: [w615 w616] -> w613
                    frame False {
                      n264 = local read "top right speed"() -> (w615:cluster{dbl, dbl, dbl})
                    }
                    frame True {
                      n265 = local read "top left speed"() -> (w616:cluster{dbl, dbl, dbl})
                    }
                  }
                }
                frame 2 {
                  n266 = case shown="False" w618 {
                    tunnel: [w619 w620] -> w617
                    frame False {
                      n267 = local read "mid line speed"() -> (w619:cluster{dbl, dbl, dbl})
                    }
                    frame True {
                      n268 = local read "mid line speed"() -> (w620:cluster{dbl, dbl, dbl})
                    }
                  }
                }
                frame 0, Default {
                  n269 = case shown="True" w622 {
                    tunnel: [w623 w624] -> w621
                    frame False {
                      n270 = local read "bottom line speed"() -> (w623:cluster{dbl, dbl, dbl})
                    }
                    frame True {
                      n271 = local read "bottom line speed"() -> (w624:cluster{dbl, dbl, dbl})
                    }
                  }
                }
              }
              n272 = Bundle("Final X"=w584, "Final Y"=w583, "Final Z"=w593) -> (w592:T8)  [unwired: 1 in]
              n273 = call "Go2XYZ (SubVI).vi"(".NET Refnum in"=w591, "Go to Coordinates"=w592, "Axis Speeds"=w582) -> (".NET Refnum out"=→"XYZ .NET Refnum out":refnum<k24>, "Final Position"=w590:T8)  [unwired: 8 in, 3 out]
              n274 = local write "Final Position"(w590) -> ()
            }
          }
        }
      }
      n275 = local read "glue time"() -> (w322:dbl)
      n276 = local read "glue time"() -> (w326:dbl)
      n277 = Divide(x=10.0 ("vX [mm]"), y=w322) -> (x/y=w323:dbl)
      n278 = Divide(x=40.0 ("vX [mm]"), y=w326) -> (x/y=w327:dbl)
      n279 = Bundle(w323, w323, w323) -> (→"top right speed":cluster{dbl, dbl, dbl})  [unwired: 1 in]
      n280 = Bundle(w327, w327, w327) -> (→"top left speed":cluster{dbl, dbl, dbl})  [unwired: 1 in]
      n281 = local read "Arduino Resource"() -> (w341:T4)
      n282 = local read "Digital I/O Pin"() -> (w340:u8)
      n283 = call <vilib>:"Digital Write Pin.vi"("Arduino Resource"=w341, "Digital I/O Pin (0)"=w340, "error in"=w342) -> ("Arduino Resource"=w346:T4, "error out"=w345:errorcluster)  [unwired: 11 in]
      n284 = call <vilib>:"Close.vi"("Arduino Resource"=w346, "error in"=w345) -> ("error out"=w344:errorcluster)  [unwired: 13 in]
      n285 = VISA Close(VISA resource name=refnum<visa-resource-name> "GlueCTRL", error in (no error)=w344) -> (error out=→"error out":errorcluster)
    }
  }
